vi "TA Main - PID - Copy.vi"() -> ()   [LabVIEW 2019]
doc: "This example demonstrates how to acquire a continuous amount of data (Waveform) using the DAQ device's internal clock. It also shows how to synchronize two devices for different device families (E Series, S Series, M Series, X Series, DSA, and SC Express), to simultaneously acquire the data.\n\nFor instructions on how to connect your signals to the DAQ device, refer to your device documentation."
uses:
  Program Files/National Instruments/LabVIEW 2019/examples/Instrument IO/Serial/support/Serial - Settings.ctl
  <vilib>/Utility/error.llb/DialogType.ctl
  <vilib>/DAQmx/read.llb/DAQmx Read (Analog 1D Wfm NChan NSamp).vi
  <vilib>/DAQmx/write.llb/DAQmx Write (Analog Wfm 1Chan NSamp).vi
  <vilib>/Instr/_visa.llb/VISA Configure Serial Port (Instr).vi
  <vilib>/DAQmx/configure/timing.llb/DAQmx Timing (Sample Clock).vi
  <vilib>/DAQmx/miscellaneous.llb/DAQmx Fill In Error Info.vi
panel:
  out "Heater Modulation":waveform(dbl)(graph)={"t0"=timestamp(28 s since 1904-01-01), "dt"=0.0001, "Y"=array[10000 elements]} caption="Waveform"
  out "Lockin chart 2":waveform(dbl)[](graph)=[{"t0"=timestamp(3657170606.5589848 s since 1904-01-01), "dt"=1.9999999999999998, "Y"=[-0.10259103252348788], "attributes"=variant("NI_ChannelName"=variant(string "Phase - Diode Voltage"), "NI_UnitDescription"=variant(string "Rad"))}, {"t0"=timestamp(3657170606.5589848 s since 1904-01-01), "dt"=1.9999999999999998, "Y"=[0.08995683165578135], "attributes"=variant("NI_ChannelName"=variant(string "Amplitude - Diode Voltage"), "NI_UnitDescription"=variant(string "Volts"))}]
  in  "Pass Logger":T1(tab)=enum."PID"
  out "CO2 chart":waveform(dbl)[](graph)=[{"t0"=timestamp(3657170606.3978887 s since 1904-01-01), "dt"=0.0, "Y"=[817.0], "attributes"=variant("NI_ChannelName"=variant(string "SCD30 CO2"), "NI_UnitDescription"=variant(string "ppm"))}, {"t0"=timestamp(3657170606.3978887 s since 1904-01-01), "dt"=0.0, "Y"=[23.97], "attributes"=variant("NI_ChannelName"=variant(string "SCD30 Temp"), "NI_UnitDescription"=variant(string "C"))}, {"t0"=timestamp(3657170606.3978887 s since 1904-01-01), "dt"=0.0, "Y"=[36.92], "attributes"=variant("NI_ChannelName"=variant(string "SCD30 Humidity"), "NI_UnitDescription"=variant(string "%"))}, {"t0"=timestamp(3657170606.3978887 s since 1904-01-01), "dt"=0.0, "Y"=[23.25], "attributes"=variant("NI_ChannelName"=variant(string "BME680 Temp"), "NI_UnitDescription"=variant(string "C"))}, {"t0"=timestamp(3657170606.3978887 s since 1904-01-01), "dt"=0.0, "Y"=[1004.82], "attributes"=variant("NI_ChannelName"=variant(string "hPa"), "NI_UnitDescription"=variant(string "BME680 Pressure"))}, {"t0"=timestamp(3657170606.3978887 s since 1904-01-01), "dt"=0.0, "Y"=[39.65], "attributes"=variant("NI_ChannelName"=variant(string "BME680 Humidity"), "NI_UnitDescription"=variant(string "%"))}, {"t0"=timestamp(3657170606.3978887 s since 1904-01-01), "dt"=0.0, "Y"=[747.02], "attributes"=variant("NI_ChannelName"=variant(string "BME680 Gas"), "NI_UnitDescription"=variant(string "KOhms"))}]
  in  "Stop":bool
  in  "Enable logging":bool caption="Enable"
  in  "File config":T2={"Filepath"=path "C:/Users/Administrator/Desktop/DAQ PAS/Test data", "Test ID"="test", "PC"="69DTQV2"}
  out "Lockin chart":waveform(dbl)[](graph)=[{"t0"=timestamp(3657170606.5589848 s since 1904-01-01), "dt"=1.9999999999999998, "Y"=[0.35840409569864184], "attributes"=variant("NI_ChannelName"=variant(string "Phase - Mic Diff"), "NI_UnitDescription"=variant(string "Rad"))}, {"t0"=timestamp(3657170606.5589848 s since 1904-01-01), "dt"=1.9999999999999998, "Y"=[0.04132909262078132], "attributes"=variant("NI_ChannelName"=variant(string "Amplitude - Mic Diff"), "NI_UnitDescription"=variant(string "Volts"))}]
  out "Lockin output 1":T3={"X"=0.01935147614577424, "Y"=0.007248713347471455, "R"=0.02066454631039066, "θ"=0.35840409569864184, "Amp"=0.04132909262078132, "dt"=1.9999999999999998, "Active channel"="Mic Diff", "Ref channel"="Heater Voltage"} {"X" format="%#_3g"; "Y" format="%#_3g"; "R" format="%#_3g"}
  out "Reference sesnsor readings":T4={"SCD30 CO2"=817.0, "SCD30 Temp (C)"=23.97, "SCD30 RH (%)"=36.92, "BME680 Temp (C) "=23.25, "BME680 Presssure (hPa)"=1004.82, "BME680 RH (%) "=39.65, "BME680 Gas (KOhms)"=747.02}
  in  "Sampling config":cluster{"Fs":dbl, "#s":dbl}={"Fs"=10000.0, "#s"=10000.0} {"Fs" format="%.2p"}
  in  "buffer size (in samples per channel)":u32
  in  "Config 1":cluster{"Ref Index":i32, "Active Index":i32}={"Ref Index"=2, "Active Index"=5}
  out "Lockin output 5":T3={"X"=-4.71813339906535, "Y"=-2.4285894180439636, "R"=5.306489360472804, "θ"=-2.66622648098918, "Amp"=10.612978720945607, "dt"=1.9999999999999998, "Active channel"="Heater Current", "Ref channel"="Heater Voltage"} {"X" format="%#_3g"; "Y" format="%#_3g"; "R" format="%#_3g"}
  out "Lockin output 6":T3={"X"=19.611612959634517, "Y"=6.527769643575472, "R"=20.66947361202239, "θ"=0.3213175235280957, "Amp"=41.33894722404478, "dt"=1.9999999999999998, "Active channel"="Heater Temperature", "Ref channel"="Heater Voltage"} {"X" format="%#_3g"; "Y" format="%#_3g"; "R" format="%#_3g"}
  out "Lockin output 4":T3={"X"=-0.22804529541896595, "Y"=-0.10244301108706262, "R"=0.24999845456183822, "θ"=-2.719385728324672, "Amp"=0.49999690912367645, "dt"=1.9999999999999998, "Active channel"="Heater Voltage", "Ref channel"="Heater Voltage"} {"X" format="%#_3g"; "Y" format="%#_3g"; "R" format="%#_3g"}
  out "Lockin output 3":T3={"X"=0.019485539557515245, "Y"=0.00689470931901729, "R"=0.02066937997234642, "θ"=0.34008918758761303, "Amp"=0.04133875994469284, "dt"=1.9999999999999998, "Active channel"="Mic Active", "Ref channel"="Heater Voltage"} {"X" format="%#_3g"; "Y" format="%#_3g"; "R" format="%#_3g"}
  out "Lockin output 2":T3={"X"=0.0003267413461158994, "Y"=-0.0008339623352990468, "R"=0.0008956858176610087, "θ"=-1.197384139538272, "Amp"=0.0017913716353220174, "dt"=1.9999999999999998, "Active channel"="Mic Ref", "Ref channel"="Heater Voltage"} {"X" format="%#_3g"; "Y" format="%#_3g"; "R" format="%#_3g"}
  in  "Config 5":cluster{"Ref Index":i32, "Active Index":i32}={"Ref Index"=2, "Active Index"=6}
  in  "Config 4":cluster{"Ref Index":i32, "Active Index":i32}={"Ref Index"=2, "Active Index"=2}
  in  "Config 3":cluster{"Ref Index":i32, "Active Index":i32}={"Ref Index"=2, "Active Index"=1}
  in  "Config 2":cluster{"Ref Index":i32, "Active Index":i32}={"Ref Index"=2, "Active Index"=0}
  in  "Config 6":cluster{"Ref Index":i32, "Active Index":i32}={"Ref Index"=2, "Active Index"=8}
  out "Lockin output 1":T3={"X"=0.01935147614577424, "Y"=0.007248713347471455, "R"=0.02066454631039066, "θ"=0.35840409569864184, "Amp"=0.04132909262078132, "dt"=1.9999999999999998, "Active channel"="Mic Diff", "Ref channel"="Heater Voltage"} {"X" format="%#_3g"; "Y" format="%#_3g"; "R" format="%#_3g"}
  in  "Config 7":cluster{"Ref Index":i32, "Active Index":i32}={"Ref Index"=2, "Active Index"=7}
  out "Lockin output 7":T3={"X"=-4.88093610591512, "Y"=-2.2652620290193846, "R"=5.3809803317000595, "θ"=-2.7070719289824767, "Amp"=10.761960663400119, "dt"=1.9999999999999998, "Active channel"="Heater Power", "Ref channel"="Heater Voltage"} {"X" format="%#_3g"; "Y" format="%#_3g"; "R" format="%#_3g"}
  in  "Config 8":cluster{"Ref Index":i32, "Active Index":i32}={"Ref Index"=2, "Active Index"=3}
  in  "Config 9":cluster{"Ref Index":i32, "Active Index":i32}={"Ref Index"=2, "Active Index"=4}
  out "Lockin output 9":T3={"X"=0.04474192624345704, "Y"=-0.004606292045853832, "R"=0.04497841582789067, "θ"=-0.10259103252348788, "Amp"=0.08995683165578135, "dt"=1.9999999999999998, "Active channel"="Diode Voltage", "Ref channel"="Heater Voltage"} {"X" format="%#_3g"; "Y" format="%#_3g"; "R" format="%#_3g"}
  out "Lockin output 8":T3={"X"=-0.04777429539770218, "Y"=-0.02309761120753558, "R"=0.0530648937080004, "θ"=-2.6912533488681167, "Amp"=0.1061297874160008, "dt"=1.9999999999999998, "Active channel"="Heater Shunt", "Ref channel"="Heater Voltage"} {"X" format="%#_3g"; "Y" format="%#_3g"; "R" format="%#_3g"}
  in  "VISA resource name 2":refnum<visa-resource-name>="COM6"
  in  "Serial Settings":T5={"baud rate"=9600, "data bits"=8, "parity"=enum."None", "stop bits"=10, "flow control"=0} {"flow control" items=["None"=0, "XON/XOFF"=1, "RTS/CTS"=2, "DTR/DSR"=4]; "stop bits" items=["1.0"=10, "1.5"=15, "2.0"=20]; "data bits" min=5 max=8 step=1; "baud rate" items=["75"=75, "110"=110, "134"=134, "150"=150, "300"=300, "600"=600, "1200"=1200, "1800"=1800, "2400"=2400, "4800"=4800, "7200"=7200, "9600"=9600, "14400"=14400, "19200"=19200, "28800"=28800, "38400"=38400, "56000"=56000, "57600"=57600, "115200"=115200, "128000"=128000, "230400"=230400]}
  out "Waveform":waveform(dbl)(graph)={"t0"=timestamp(3657170606.558974 s since 1904-01-01), "dt"=9.999999999999999e-05, "Y"=array[20001 elements], "attributes"=variant("NI_ChannelName"=variant(string "Mic Diff"), "NI_UnitDescription"=variant(string "Volts"))}
  in  "Config":T6={"Active Index"=1, "Ref Index"=0, "Gain"=1.0, "Channel name"="Mic Diff", "Enable"=TRUE, "Offset"=0.0}
  out "Channel names":T7={"Active channel"="Mic Active", "Ref channel"="Mic Ref"}
  in  "Waveform Config":T8={"Frequency"=10.0, "Voltage (V)"=1.0, "Signal type"=enum."Sine Wave", "Square wave duty cycle (%)"=50.0, "Offset (V)"=0.0, "DC shift"=TRUE} {"Square wave duty cycle (%)" format="%0.2f"}
  in  "Output range":cluster{"output high":dbl, "output low":dbl}={"output high"=1.6, "output low"=0.0}
  in  "Channel config":T9={"physical channels"="Dev1/ao0", "name to assign"="Heater Voltage"}
  in  "Config":T10={"Voltage channel index"=2, "Shunt channel index"=3, "Shunt resistance"=10}
  out "Channel names":T11={"Voltage channel name"="Heater Voltage", "Shunt channel name"="Heater Shunt"}
  out "Microphone Waveform":waveform(dbl)[](graph)=[{"t0"=timestamp(3657170606.558963 s since 1904-01-01), "dt"=9.999999999999999e-05, "Y"=array[20001 elements], "attributes"=variant("NI_ChannelName"=variant(string "Mic Ref"), "NI_UnitDescription"=variant(string "Volts"))}, {"t0"=timestamp(3657170606.558974 s since 1904-01-01), "dt"=9.999999999999999e-05, "Y"=array[20001 elements], "attributes"=variant("NI_ChannelName"=variant(string "Mic Active"), "NI_UnitDescription"=variant(string "Volts"))}, {"t0"=timestamp(3657170606.5589848 s since 1904-01-01), "dt"=9.999999999999999e-05, "Y"=array[20001 elements], "attributes"=variant("NI_ChannelName"=variant(string "Heater Voltage"), "NI_UnitDescription"=variant(string "Volts"))}, {"t0"=timestamp(3657170606.5589957 s since 1904-01-01), "dt"=9.999999999999999e-05, "Y"=array[20001 elements], "attributes"=variant("NI_ChannelName"=variant(string "Heater Shunt"), "NI_UnitDescription"=variant(string "Volts"))}, {"t0"=timestamp(3657170606.5590067 s since 1904-01-01), "dt"=9.999999999999999e-05, "Y"=array[20001 elements], "attributes"=variant("NI_ChannelName"=variant(string "Diode Voltage"), "NI_UnitDescription"=variant(string "Volts"))}, {"t0"=timestamp(3657170606.558974 s since 1904-01-01), "dt"=9.999999999999999e-05, "Y"=array[20001 elements], "attributes"=variant("NI_ChannelName"=variant(string "Mic Diff"), "NI_UnitDescription"=variant(string "Volts"))}, {"t0"=timestamp(3657170606.5589957 s since 1904-01-01), "dt"=9.999999999999999e-05, "Y"=array[20001 elements], "attributes"=variant("NI_ChannelName"=variant(string "Heater Current"), "NI_UnitDescription"=variant(string "mA"))}, {"t0"=timestamp(3657170606.5589848 s since 1904-01-01), "dt"=9.999999999999999e-05, "Y"=array[20001 elements], "attributes"=variant("NI_ChannelName"=variant(string "Heater Power"), "NI_UnitDescription"=variant(string "mW"))}, {"t0"=timestamp(3657170606.558974 s since 1904-01-01), "dt"=9.999999999999999e-05, "Y"=array[20001 elements], "attributes"=variant("NI_ChannelName"=variant(string "Heater Temperature"), "NI_UnitDescription"=variant(string "degC"))}]
  out "Heater Waveform":waveform(dbl)[](graph)=[{"t0"=timestamp(3657170606.558963 s since 1904-01-01), "dt"=9.999999999999999e-05, "Y"=array[20001 elements], "attributes"=variant("NI_ChannelName"=variant(string "Mic Ref"), "NI_UnitDescription"=variant(string "Volts"))}, {"t0"=timestamp(3657170606.558974 s since 1904-01-01), "dt"=9.999999999999999e-05, "Y"=array[20001 elements], "attributes"=variant("NI_ChannelName"=variant(string "Mic Active"), "NI_UnitDescription"=variant(string "Volts"))}, {"t0"=timestamp(3657170606.5589848 s since 1904-01-01), "dt"=9.999999999999999e-05, "Y"=array[20001 elements], "attributes"=variant("NI_ChannelName"=variant(string "Heater Voltage"), "NI_UnitDescription"=variant(string "Volts"))}, {"t0"=timestamp(3657170606.5589957 s since 1904-01-01), "dt"=9.999999999999999e-05, "Y"=array[20001 elements], "attributes"=variant("NI_ChannelName"=variant(string "Heater Shunt"), "NI_UnitDescription"=variant(string "Volts"))}, {"t0"=timestamp(3657170606.5590067 s since 1904-01-01), "dt"=9.999999999999999e-05, "Y"=array[20001 elements], "attributes"=variant("NI_ChannelName"=variant(string "Diode Voltage"), "NI_UnitDescription"=variant(string "Volts"))}, {"t0"=timestamp(3657170606.558974 s since 1904-01-01), "dt"=9.999999999999999e-05, "Y"=array[20001 elements], "attributes"=variant("NI_ChannelName"=variant(string "Mic Diff"), "NI_UnitDescription"=variant(string "Volts"))}, {"t0"=timestamp(3657170606.5589957 s since 1904-01-01), "dt"=9.999999999999999e-05, "Y"=array[20001 elements], "attributes"=variant("NI_ChannelName"=variant(string "Heater Current"), "NI_UnitDescription"=variant(string "mA"))}, {"t0"=timestamp(3657170606.5589848 s since 1904-01-01), "dt"=9.999999999999999e-05, "Y"=array[20001 elements], "attributes"=variant("NI_ChannelName"=variant(string "Heater Power"), "NI_UnitDescription"=variant(string "mW"))}, {"t0"=timestamp(3657170606.558974 s since 1904-01-01), "dt"=9.999999999999999e-05, "Y"=array[20001 elements], "attributes"=variant("NI_ChannelName"=variant(string "Heater Temperature"), "NI_UnitDescription"=variant(string "degC"))}]
  out "Diode Waveform":waveform(dbl)[](graph)=[{"t0"=timestamp(3657170606.558963 s since 1904-01-01), "dt"=9.999999999999999e-05, "Y"=array[20001 elements], "attributes"=variant("NI_ChannelName"=variant(string "Mic Ref"), "NI_UnitDescription"=variant(string "Volts"))}, {"t0"=timestamp(3657170606.558974 s since 1904-01-01), "dt"=9.999999999999999e-05, "Y"=array[20001 elements], "attributes"=variant("NI_ChannelName"=variant(string "Mic Active"), "NI_UnitDescription"=variant(string "Volts"))}, {"t0"=timestamp(3657170606.5589848 s since 1904-01-01), "dt"=9.999999999999999e-05, "Y"=array[20001 elements], "attributes"=variant("NI_ChannelName"=variant(string "Heater Voltage"), "NI_UnitDescription"=variant(string "Volts"))}, {"t0"=timestamp(3657170606.5589957 s since 1904-01-01), "dt"=9.999999999999999e-05, "Y"=array[20001 elements], "attributes"=variant("NI_ChannelName"=variant(string "Heater Shunt"), "NI_UnitDescription"=variant(string "Volts"))}, {"t0"=timestamp(3657170606.5590067 s since 1904-01-01), "dt"=9.999999999999999e-05, "Y"=array[20001 elements], "attributes"=variant("NI_ChannelName"=variant(string "Diode Voltage"), "NI_UnitDescription"=variant(string "Volts"))}, {"t0"=timestamp(3657170606.558974 s since 1904-01-01), "dt"=9.999999999999999e-05, "Y"=array[20001 elements], "attributes"=variant("NI_ChannelName"=variant(string "Mic Diff"), "NI_UnitDescription"=variant(string "Volts"))}, {"t0"=timestamp(3657170606.5589957 s since 1904-01-01), "dt"=9.999999999999999e-05, "Y"=array[20001 elements], "attributes"=variant("NI_ChannelName"=variant(string "Heater Current"), "NI_UnitDescription"=variant(string "mA"))}, {"t0"=timestamp(3657170606.5589848 s since 1904-01-01), "dt"=9.999999999999999e-05, "Y"=array[20001 elements], "attributes"=variant("NI_ChannelName"=variant(string "Heater Power"), "NI_UnitDescription"=variant(string "mW"))}, {"t0"=timestamp(3657170606.558974 s since 1904-01-01), "dt"=9.999999999999999e-05, "Y"=array[20001 elements], "attributes"=variant("NI_ChannelName"=variant(string "Heater Temperature"), "NI_UnitDescription"=variant(string "degC"))}]
  in  "Channel 4 config":T12={"Channel"="Dev1/ai3", "Vmax"=0.5, "Vmin"=0.0, "name to assign"="Heater Shunt", "input terminal configuration"=10106} {"input terminal configuration" items=["Default"=-1, "RSE"=10083, "NRSE"=10078, "Differential"=10106, "Pseudodifferential"=12529]; "Vmin" format="%0.2f"; "Vmax" format="%0.2f"}
  in  "Channel 3 config":T12={"Channel"="Dev1/ai2", "Vmax"=3.0, "Vmin"=0.0, "name to assign"="Heater Voltage", "input terminal configuration"=10083} {"input terminal configuration" items=["Default"=-1, "RSE"=10083, "NRSE"=10078, "Differential"=10106, "Pseudodifferential"=12529]; "Vmin" format="%0.2f"; "Vmax" format="%0.2f"}
  in  "Channel 2 config":T12={"Channel"="Dev1/ai1", "Vmax"=3.0, "Vmin"=-3.0, "name to assign"="Mic Active", "input terminal configuration"=10083} {"input terminal configuration" items=["Default"=-1, "RSE"=10083, "NRSE"=10078, "Differential"=10106, "Pseudodifferential"=12529]; "Vmin" format="%0.2f"; "Vmax" format="%0.2f"}
  in  "Channel 1 config":T12={"Channel"="Dev1/ai0", "Vmax"=3.0, "Vmin"=-3.0, "name to assign"="Mic Ref", "input terminal configuration"=10083} {"input terminal configuration" items=["Default"=-1, "RSE"=10083, "NRSE"=10078, "Differential"=10106, "Pseudodifferential"=12529]; "Vmin" format="%0.2f"; "Vmax" format="%0.2f"}
  in  "Channel 5 config":T12={"Channel"="Dev1/ai4", "Vmax"=1.0, "Vmin"=0.0, "name to assign"="Diode Voltage", "input terminal configuration"=10083} {"input terminal configuration" items=["Default"=-1, "RSE"=10083, "NRSE"=10078, "Differential"=10106, "Pseudodifferential"=12529]; "Vmin" format="%0.2f"; "Vmax" format="%0.2f"}
  out "Boolean":bool
  out "PID output":dbl format="%.2f"
  in  "reinitialize? (F)":bool
  in  "auto? (F)":bool
  in  "PID gains":T13={"proportional gain (Kc)"=0.0125026, "integral time (Ti, min)"=2.0, "derivative time (Td, min)"=0.0} {"derivative time (Td, min)" format="%.6f"; "integral time (Ti, min)" format="%.6f"; "proportional gain (Kc)" format="%.6f"}
  in  "Temp config":T14={"Channel Index"=4, "TC"=0.001, "Channel name"="Heater Temperature", "25C Voltage"=0.80857} {"25C Voltage" format="%.5f"; "TC" format="%#_6f"}
  out "Sensor channel":string="Mic Active"
  in  "Store":bool
  in  "setpoint":dbl
  # "PAS Logger"
  # "(ppm)"
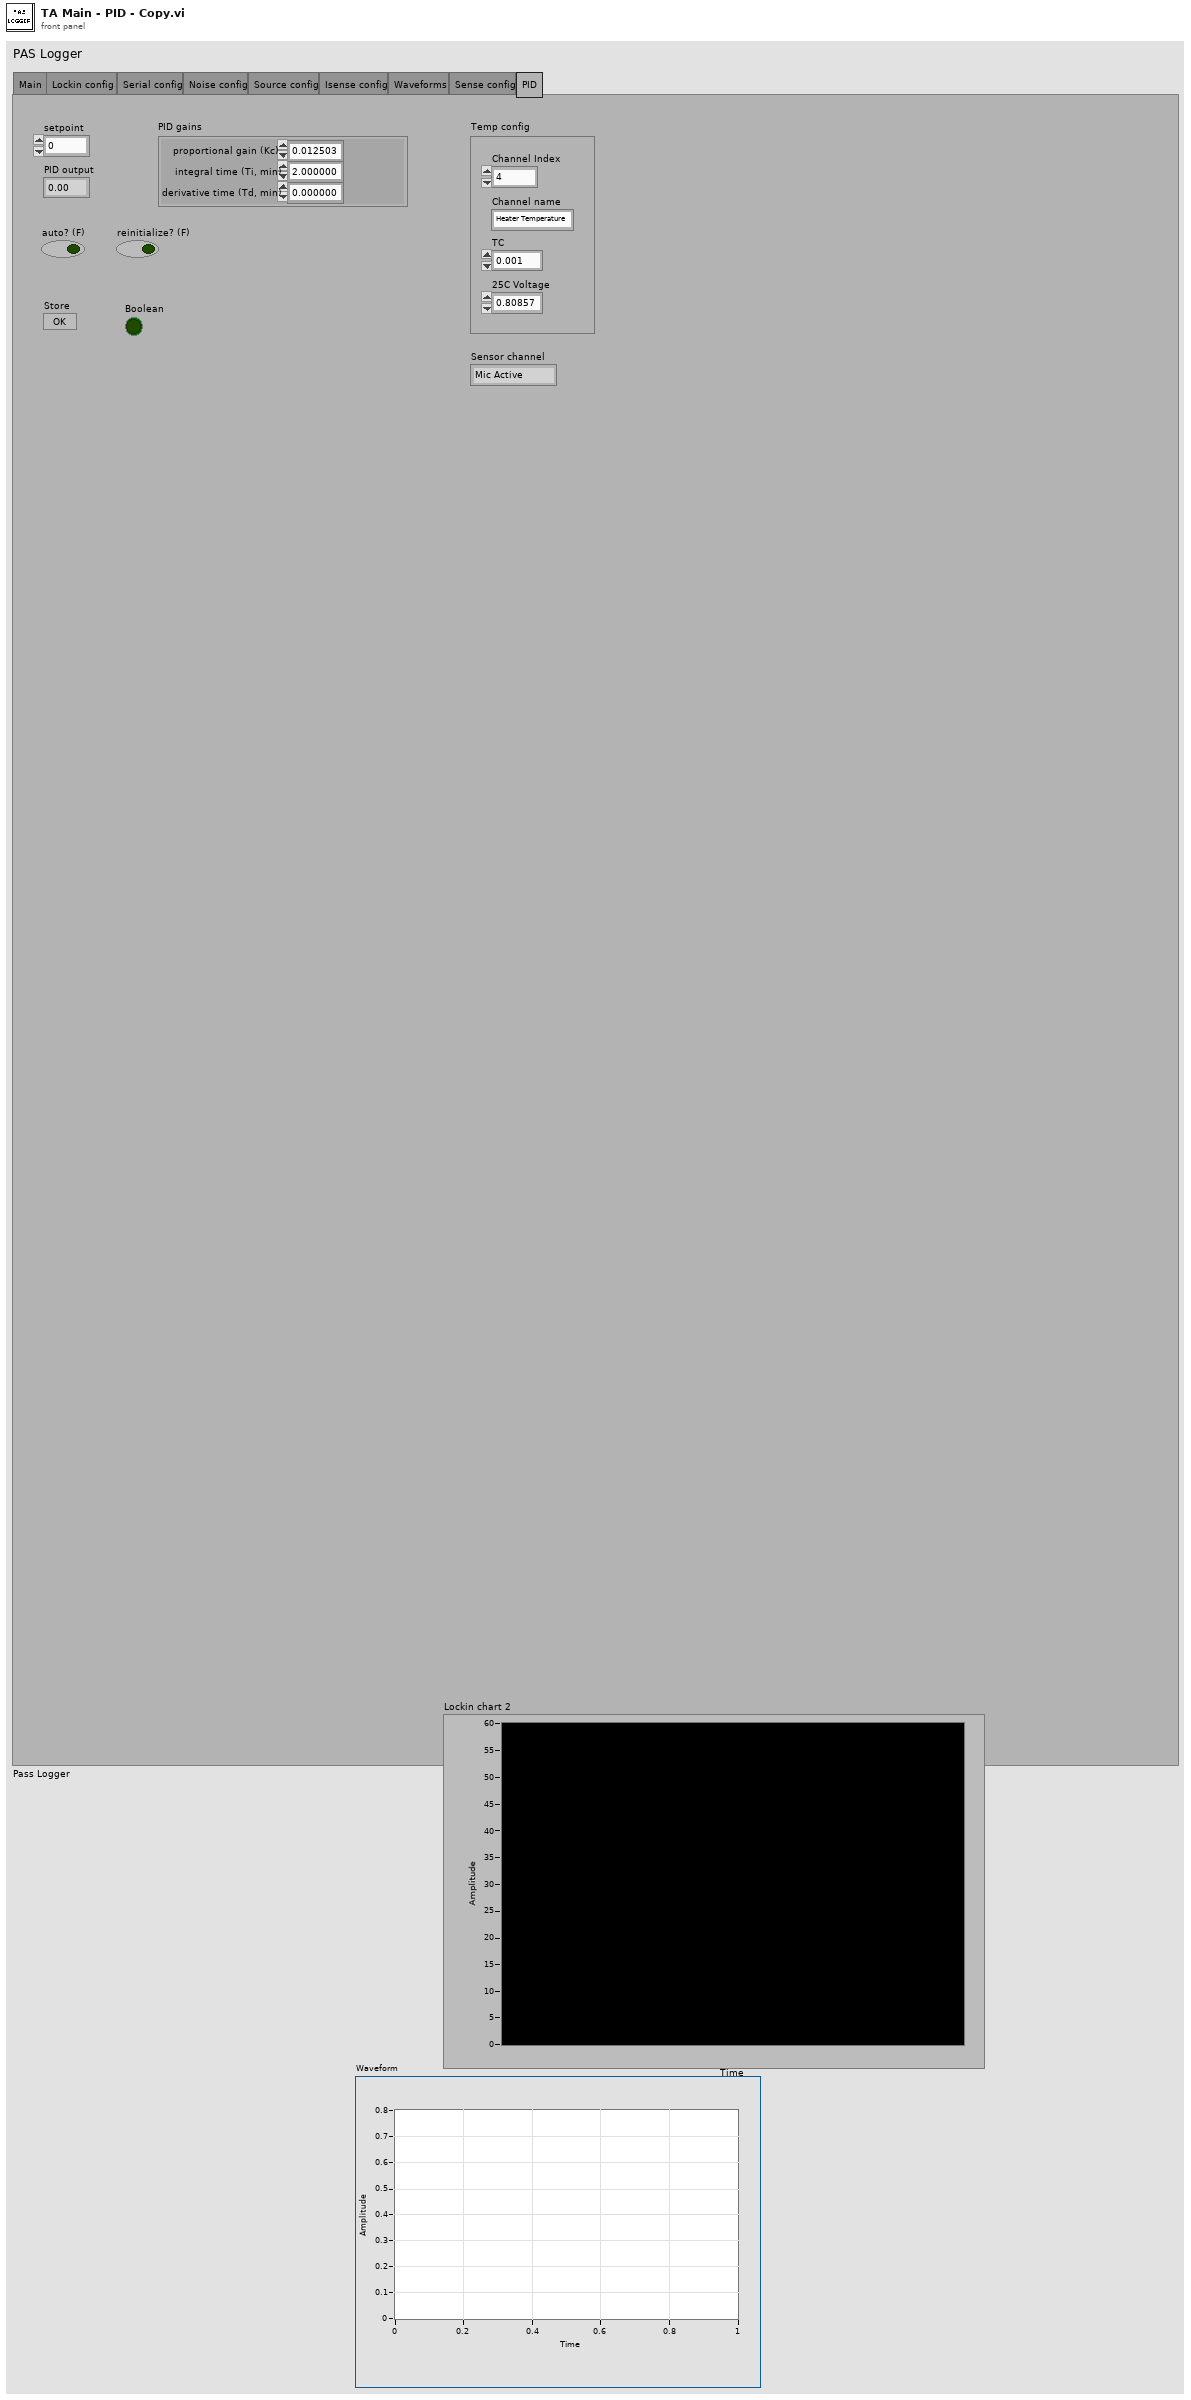
[diagram p1: front panel]
types:
  T1 = enum32{"Main", "Lockin config", "Serial config", "Noise config", "Source config", "Isense config", "Waveforms", "Sense config", "PID"}
  T2 = cluster{"Filepath":path, "Test ID":string, "PC":string}
  T3 = cluster{"X":dbl, "Y":dbl, "R":dbl, "θ":dbl, "Amp":dbl, "dt":dbl, "Active channel":string, "Ref channel":string}
  T4 = cluster{"SCD30 CO2":dbl, "SCD30 Temp (C)":dbl, "SCD30 RH (%)":dbl, "BME680 Temp (C) ":dbl, "BME680 Presssure (hPa)":dbl, "BME680 RH (%) ":dbl, "BME680 Gas (KOhms)":dbl}
  T5 = typedef "Serial - Settings.ctl" = cluster{"baud rate":u32, "data bits":u16, "parity":enum16{"None", "Odd", "Even", "Mark", "Space"}, "stop bits":u16, "flow control":u16}
  T6 = cluster{"Active Index":i32, "Ref Index":i32, "Gain":dbl, "Channel name":string, "Enable":bool, "Offset":dbl}
  T7 = cluster{"Active channel":string, "Ref channel":string}
  T8 = cluster{"Frequency":dbl, "Voltage (V)":dbl, "Signal type":enum16{"Sine Wave", "Triangle Wave", "Square Wave", "Sawtooth Wave"}, "Square wave duty cycle (%)":dbl, "Offset (V)":dbl, "DC shift":bool}
  T9 = cluster{"physical channels":tag, "name to assign":string}
  T10 = cluster{"Voltage channel index":i32, "Shunt channel index":i32, "Shunt resistance":i32}
  T11 = cluster{"Voltage channel name":string, "Shunt channel name":string}
  T12 = cluster{"Channel":tag, "Vmax":dbl, "Vmin":dbl, "name to assign":string, "input terminal configuration":i32}
  T13 = cluster{"proportional gain (Kc)":dbl, "integral time (Ti, min)":dbl, "derivative time (Td, min)":dbl}
  T14 = cluster{"Channel Index":i32, "TC":dbl, "Channel name":string, "25C Voltage":dbl}
  T15 = typedef "DialogType.ctl" = u16
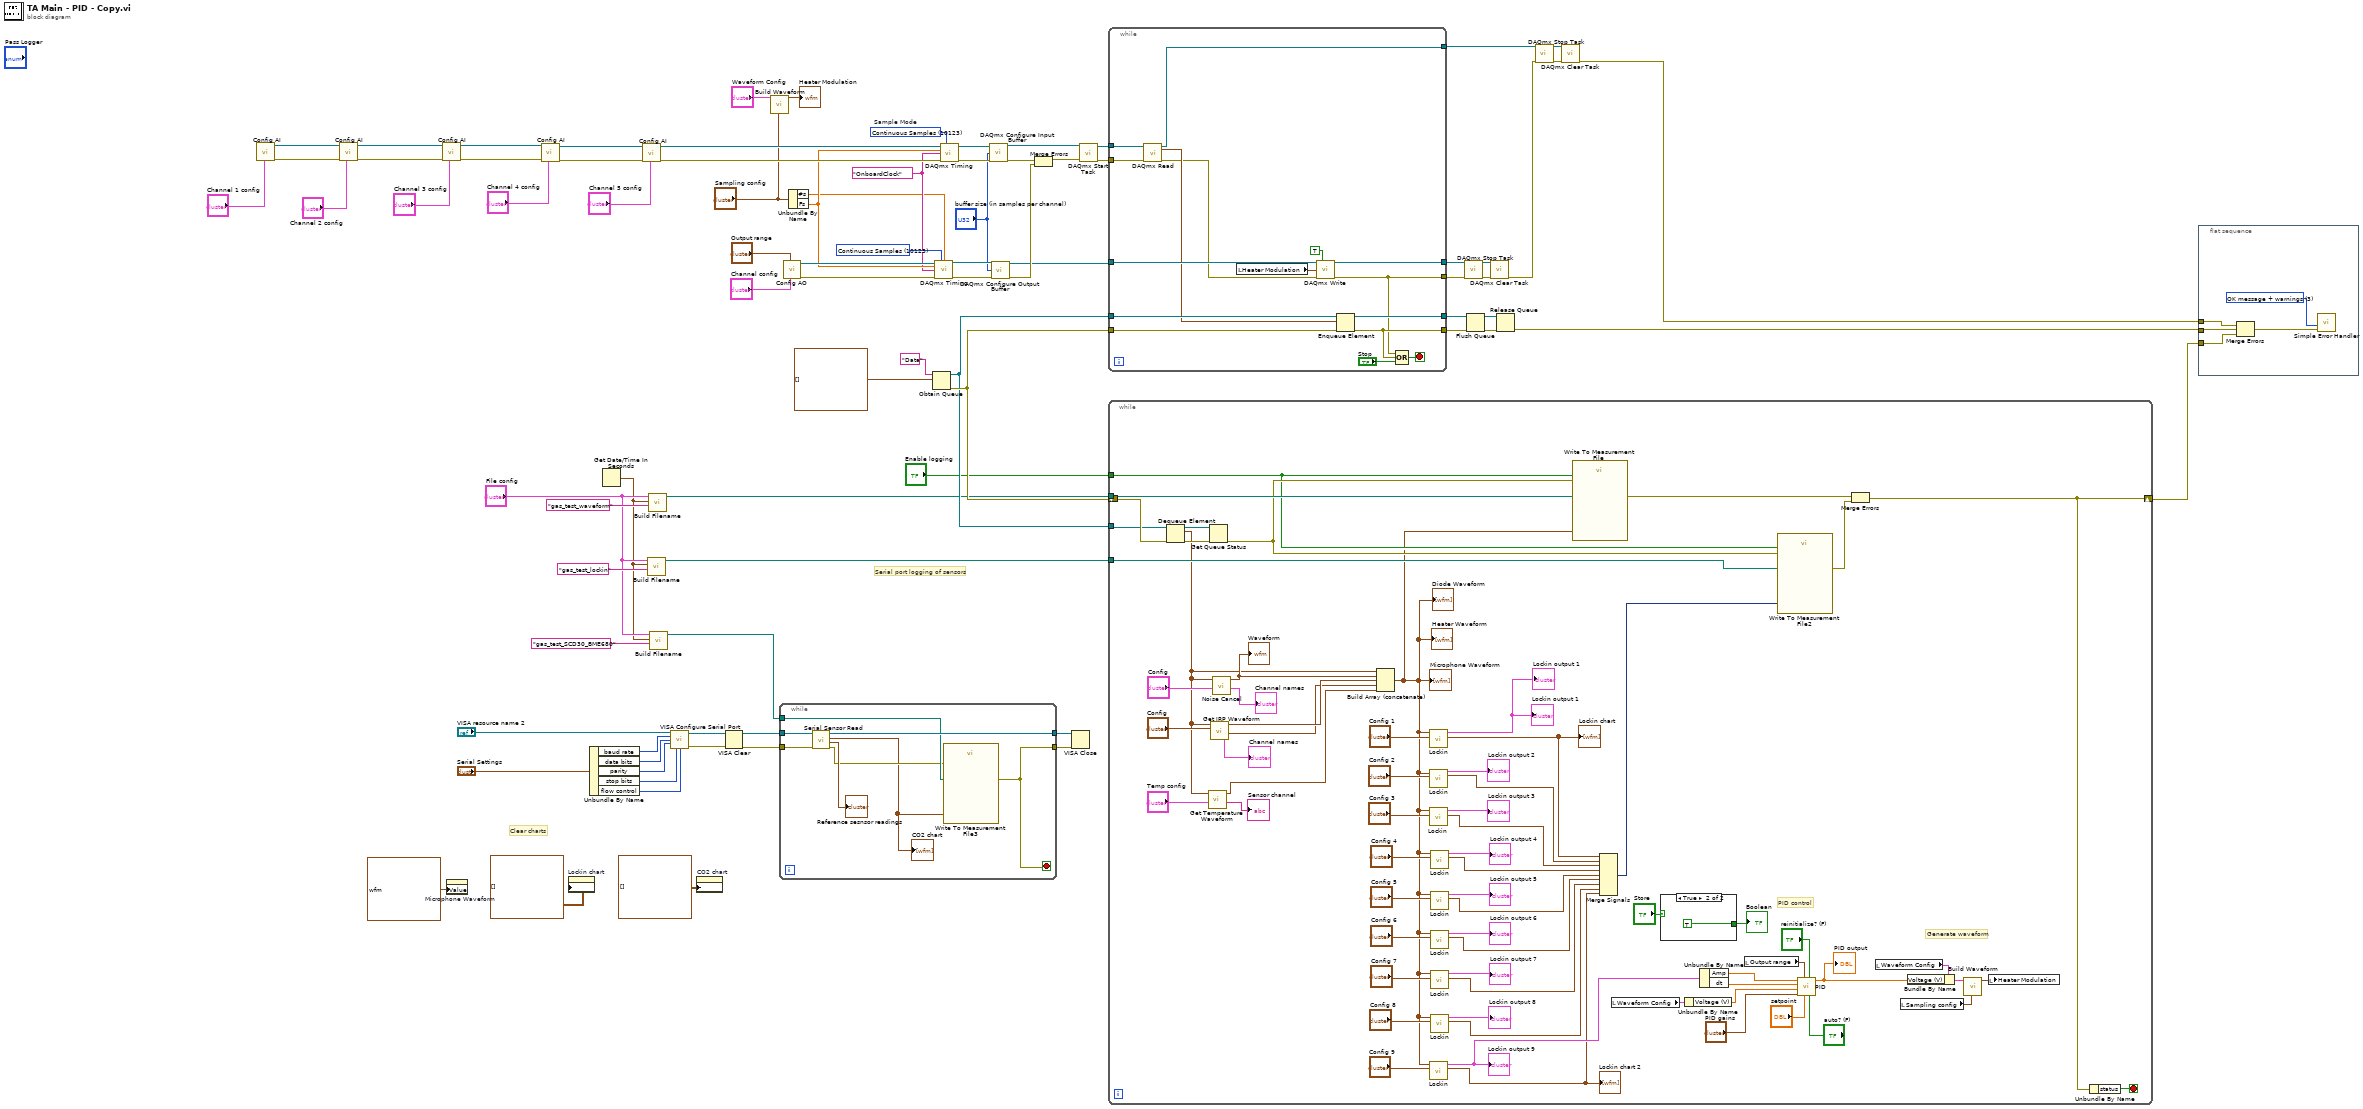
[diagram p0: block diagram]
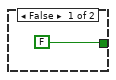
[diagram p2: hidden frame]
diagram:
  w32 = 10123 items=["Finite Samples"=10178, "Continuous Samples"=10123, "Hardware Timed Single Point"=12522] ("sample mode")
  w26 = tag "OnboardClock" ("source")
  w81 = 10123 items=["Finite Samples"=10178, "Continuous Samples"=10123, "Hardware Timed Single Point"=12522]  # Sample Mode
  # "Clear charts"
  # "Serial port logging of sensors"
  n1 = call "Config AI.vi"("Channel config"="Channel 1 config") -> ("error out"=w80:errorcluster, "task out"=w79:refnum<k21>)  [unwired: 9 in]
  n2 = call "Config AI.vi"("Channel config"="Channel 2 config", "error in"=w80, "task in"=w79) -> ("error out"=w37:errorcluster, "task out"=w36:refnum<k21>)  [unwired: 7 in]
  n3 = call "Config AI.vi"("Channel config"="Channel 3 config", "error in"=w37, "task in"=w36) -> ("error out"=w68:errorcluster, "task out"=w67:refnum<k21>)  [unwired: 7 in]
  n4 = property on="Microphone Waveform" class="WFGraph (strict)"("Value"=waveform(dbl)[] [{"t0"=timestamp(3651561790.263236 s since 1904-01-01), "dt"=0.001, "Y"=array[2000 elements], "attributes"=variant("NI_ChannelName"=variant(string "Mic Active"), "NI_UnitDescription"=variant(string "Volts"))}, {"t0"=timestamp(3651561790.263247 s since 1904-01-01), "dt"=0.001, "Y"=array[2000 elements], "attributes"=variant("NI_ChannelName"=variant(string "Mic Ref"), "NI_UnitDescription"=variant(string "Volts"))}, {"t0"=timestamp(3651561790.263258 s since 1904-01-01), "dt"=0.001, "Y"=array[2000 elements], "attributes"=variant("NI_ChannelName"=variant(string "Diode Heater"), "NI_UnitDescription"=variant(string "Volts"))}, {"t0"=timestamp(3651561790.263269 s since 1904-01-01), "dt"=0.001, "Y"=array[2000 elements], "attributes"=variant("NI_ChannelName"=variant(string "Diode Amb"), "NI_UnitDescription"=variant(string "Volts"))}, {"t0"=timestamp(3651561790.26328 s since 1904-01-01), "dt"=0.001, "Y"=array[2000 elements], "attributes"=variant("NI_ChannelName"=variant(string "Heater Shunt"), "NI_UnitDescription"=variant(string "Volts"))}, {"t0"=timestamp(3651561790.2632914 s since 1904-01-01), "dt"=0.001, "Y"=array[2000 elements], "attributes"=variant("NI_ChannelName"=variant(string "Heater V"), "NI_UnitDescription"=variant(string "Volts"))}, {"t0"=timestamp(3651561790.263247 s since 1904-01-01), "dt"=0.001, "Y"=array[2000 elements], "attributes"=variant("NI_ChannelName"=variant(string "Mic Diff"), "NI_UnitDescription"=variant(string "Volts"))}, {"t0"=timestamp(3651561790.26328 s since 1904-01-01), "dt"=0.001, "Y"=array[2000 elements], "attributes"=variant("NI_ChannelName"=variant(string "Heater Current"), "NI_UnitDescription"=variant(string "Amps"))}] ("Waveform")) -> ()  [unwired: 2 in, 2 out]
  n5 = call "Config AI.vi"("Channel config"="Channel 4 config", "error in"=w68, "task in"=w67) -> ("error out"=w34:errorcluster, "task out"=w33:refnum<k21>)  [unwired: 7 in]
  n6 = property on="Lockin chart" class="WFChart (strict)"("History Data"=waveform(dbl)[][] []) -> ()  [unwired: 2 in, 2 out]
  n7 = Unbundle By Name("Serial Settings") -> ("baud rate"=w52:u32, "data bits"=w51:u16, "parity"=w50:enum16{"None", "Odd", "Even", "Mark", "Space"}, "stop bits"=w49:u16, "flow control"=w48:u16)
  n8 = Get Date/Time In Seconds() -> (seconds since 1Jan1904=w55:timestamp)
  n9 = call "Config AI.vi"("Channel config"="Channel 5 config", "error in"=w34, "task in"=w33) -> ("error out"=w29:errorcluster, "task out"=w28:refnum<k21>)  [unwired: 7 in]
  n10 = call "Build Filename.vi"("Test type"="gas_test_lockin" ("File Descriptor"), "time stamp"=w55, "File config"="File config") -> ("appended path"=w58:path)  [unwired: 8 in]
  n11 = call "Build Filename.vi"("Test type"="gas_test_waveform" ("File type"), "time stamp"=w55, "File config"="File config") -> ("appended path"=w60:path)  [unwired: 8 in]
  n12 = call "Build Filename.vi"("Test type"="gas_test_SCD30_BME680" ("File Descriptor"), "time stamp"=w55, "File config"="File config") -> ("appended path"=w41:path)  [unwired: 8 in]
  n13 = call-poly "VISA Configure Serial Port"("VISA resource name"="VISA resource name 2", "baud rate (9600)"=w52, "data bits (8)"=w51, "parity (0:none)"=w50, "stop bits (10: 1 bit)"=w49, "flow control (0:none)"=w48) -> ("VISA resource name out"=w46:refnum<visa-resource-name>, "error out"=w47:errorcluster)  [unwired: 3 in, 5 out]
  n14 = property on="CO2 chart" class="WFChart (strict)"("History Data"=waveform(dbl)[][] []) -> ()  [unwired: 2 in, 2 out]
  n15 = VISA Clear(VISA resource name=w46, error in (no error)=w47) -> (VISA resource name out=w45:refnum<visa-resource-name>, error out=w44:errorcluster)
  n16 = call "Build Waveform.vi"("sampling config"="Sampling config", "Config"="Waveform Config") -> ("Waveform"=→"Heater Modulation":waveform(dbl))  [unwired: 8 in, 1 out]
  n17 = while {
    tunnel: w45 -> [w91]
    tunnel: w44 -> [w90]
    tunnel: [w85] -> w43
    tunnel: [w89] -> w42
    tunnel: w41 -> [w87]
    stop <- w85 stop-if-true
    n18 = call "Serial Sensor Read.vi"("error in (no error)"=w90, "VISA resource name"=w91) -> ("error out"=w86:errorcluster, "Readings"=→"Reference sesnsor readings":T4, "appended array"=w84:waveform(dbl)[], "VISA resource name out"=w89:refnum<visa-resource-name>)  [unwired: 6 in]
    "CO2 chart" <- w84
    n19 = call "Write To Measurement File3"("Signals"=w84, "error in (no error)"=w86, "Filename"=w87) -> ("error out"=w85:errorcluster)  [unwired: 14 in, 2 out]
  }
  n20 = call "Config AO.vi"("Channel config"="Channel config", "Output range"="Output range") -> ("error out"=w31:errorcluster, "task out"=w30:refnum<k21>)  [unwired: 8 in]
  n21 = Unbundle By Name("Sampling config") -> ("#s"=w15:dbl, "Fs"=w27:dbl)
  n22 = Obtain Queue(name (unnamed)="Data" ("名前（名前なし）"), element data type=waveform(dbl)[] [] ("data")) -> (queue out=w71:refnum<queue>, error out=w72:errorcluster)  [unwired: 3 in, 1 out]
  n23 = call-poly <vilib>:"DAQmx Timing.vi"("task/channels in"=w30, "sample mode"=w32, "samples per channel"=w15, "rate"=w27, "source"=w26, "error in"=w31) -> ("task out"=w5:refnum<k21>, "error out"=w4:errorcluster)  [unwired: 8 in]
  n24 = call-poly <vilib>:"DAQmx Timing.vi"("task/channels in"=w28, "sample mode"=w81, "rate"=w27, "source"=w26, "error in"=w29) -> ("task out"=w7:refnum<k21>, "error out"=w9:errorcluster)  [unwired: 9 in]
  n25 = call <vilib>:"DAQmx Configure Input Buffer.vi"("task/channels in"=w7, "buffer size (in samples per channel)"="buffer size (in samples per channel)", "error in"=w9) -> ("task out"=w6:refnum<k21>, "error out"=w8:errorcluster)  [unwired: 11 in]
  n26 = call <vilib>:"DAQmx Configure Output Buffer.vi"("task/channels in"=w5, "buffer size (in samples per channel)"="buffer size (in samples per channel)", "error in"=w4) -> ("task out"=w2:refnum<k21>, "error out"=w3:errorcluster)  [unwired: 11 in]
  n27 = Merge Errors(w8, w3) -> (w11:errorcluster)
  n28 = VISA Close(VISA resource name=w42, error in (no error)=w43) -> ()  [unwired: 1 out]
  n29 = call <vilib>:"DAQmx Start Task.vi"("task/channels in"=w6, "error in"=w11) -> ("task out"=w25:refnum<k21>, "error out"=w24:errorcluster)  [unwired: 12 in]
  n30 = while {
    tunnel: w71 -> [w158]
    shift-right: [w149] -> w70
    shift-left: w72 -> [w159]
    tunnel: w60 -> [w157]
    tunnel: "Enable logging" -> [w153]
    tunnel: w58 -> [w152]
    stop <- w145 stop-if-true
    # "Generate waveform"
    # "PID control"
    n31 = Dequeue Element(queue=w158, error in (no error)=w159) -> (queue out=w155:refnum<queue>, element=w114:waveform(dbl)[], error out=w156:errorcluster)  [unwired: 1 in, 1 out]
    n32 = call "Get Temperature Waveform.vi"("Config"="Temp config", "array"=w114) -> ("Channel name"=→"Sensor channel":string, "waveform out"=w111:waveform(dbl))  [unwired: 8 in]
    n33 = Get Queue Status(queue=w155, error in (no error)=w156) -> (error out=w154:errorcluster)  [unwired: 1 in, 7 out]
    n34 = call "Get IRP Waveform.vi"("Channel config"="Config", "array"=w114) -> ("Power waveform out"=w112:waveform(dbl), "Current waveform out"=w125:waveform(dbl), "Channel names"=→"Channel names":T11)  [unwired: 6 in, 1 out]
    n35 = call "Noise Cancel.vi"("Config"="Config", "array"=w114) -> ("Channel names"=→"Channel names":T7, "waveform out"=w147:waveform(dbl))  [unwired: 8 in]
    "Waveform" <- w147
    n36 = Build Array (concatenate)(w114, w147, w125, w112, w111) -> (w116:waveform(dbl)[])
    "Microphone Waveform" <- w116
    "Heater Waveform" <- w116
    "Diode Waveform" <- w116
    n37 = call "Lockin.vi"("Config"="Config 3", "array"=w116) -> ("Output waveform"=w142:waveform(dbl)[], "Lockin output"=→"Lockin output 3":T3)  [unwired: 8 in]
    n38 = call "Lockin.vi"("Config"="Config 1", "array"=w116) -> ("Output waveform"=w127:waveform(dbl)[], "Lockin output"=→"Lockin output 1" →"Lockin output 1":T3)  [unwired: 8 in]
    "Lockin chart" <- w127
    n39 = call "Lockin.vi"("Config"="Config 2", "array"=w116) -> ("Output waveform"=w143:waveform(dbl)[], "Lockin output"=→"Lockin output 2":T3)  [unwired: 8 in]
    n40 = call "Lockin.vi"("Config"="Config 9", "array"=w116) -> ("Output waveform"=w102:waveform(dbl)[], "Lockin output"=w104:T3)  [unwired: 8 in]
    "Lockin output 9" <- w104
    "Lockin chart 2" <- w102
    n41 = call "Lockin.vi"("Config"="Config 4", "array"=w116) -> ("Output waveform"=w141:waveform(dbl)[], "Lockin output"=→"Lockin output 4":T3)  [unwired: 8 in]
    n42 = call "Lockin.vi"("Config"="Config 8", "array"=w116) -> ("Output waveform"=w118:waveform(dbl)[], "Lockin output"=→"Lockin output 8":T3)  [unwired: 8 in]
    n43 = call "Lockin.vi"("Config"="Config 5", "array"=w116) -> ("Output waveform"=w140:waveform(dbl)[], "Lockin output"=→"Lockin output 5":T3)  [unwired: 8 in]
    n44 = call "Lockin.vi"("Config"="Config 6", "array"=w116) -> ("Output waveform"=w139:waveform(dbl)[], "Lockin output"=→"Lockin output 6":T3)  [unwired: 8 in]
    n45 = call "Lockin.vi"("Config"="Config 7", "array"=w116) -> ("Output waveform"=w121:waveform(dbl)[], "Lockin output"=→"Lockin output 7":T3)  [unwired: 8 in]
    n46 = call "Write To Measurement File"("Signals"=w116, "Enable"=w153, "error in (no error)"=w154, "Filename"=w157) -> ("error out"=w150:errorcluster)  [unwired: 13 in, 2 out]
    n47 = Merge Signals(w127, w143, w142, w141, w140, w139, w121, w118, w102) -> (w138:dynamicdata)
    n48 = local read "Waveform Config"() -> (w101:T8)
    n49 = case shown="True" "Store" {
      tunnel: [FALSE TRUE ("Boolean")] -> w92
      frame False {
      }
      frame True {
      }
    }
    "Boolean" <- w92
    n50 = Unbundle By Name(w101) -> ("Voltage (V)"=w100:dbl)
    n51 = Unbundle By Name(w104) -> ("Amp"=w109:dbl, "dt"=w108:dbl)
    n52 = local read "Output range"() -> (w106:cluster{"output high":dbl, "output low":dbl})
    n53 = call "Write To Measurement File2"("Signals"=w138, "Enable"=w153, "error in (no error)"=w154, "Filename"=w152) -> ("error out"=w151:errorcluster)  [unwired: 13 in, 2 out]
    n54 = call "PID.vi"("auto? (F)"="auto? (F)", "reinitialize? (F)"="reinitialize? (F)", "setpoint"="setpoint", "output range"=w106, "PID gains"="PID gains", "manual control"=w100, "dt (s)"=w108, "input"=w109) -> ("output"=w98:dbl)  [unwired: 3 in]
    "PID output" <- w98
    n55 = Merge Errors(w150, w151) -> (w149:errorcluster)
    n56 = local read "Waveform Config"() -> (w99:T8)
    n57 = local read "Sampling config"() -> (w96:cluster{"Fs":dbl, "#s":dbl})
    n58 = Bundle By Name(cluster=w99, "Voltage (V)"=w98) -> (w97:T8)
    n59 = call "Build Waveform.vi"("sampling config"=w96, "Config"=w97) -> ("Waveform"=w95:waveform(dbl))  [unwired: 8 in, 1 out]
    n60 = local write "Heater Modulation"(w95) -> ()
    n61 = Unbundle By Name(w149) -> ("status"=w145:bool)
  }
  n62 = while {
    tunnel: [w176] -> w76
    tunnel: [w172] -> w75
    tunnel: w71 -> [w175]
    tunnel: w72 -> [w174]
    tunnel: w25 -> [w171]
    tunnel: w24 -> [w170]
    tunnel: w2 -> [w169]
    tunnel: [w168] -> w22
    tunnel: [w166] -> w19
    tunnel: [w167] -> w18
    stop <- w177 stop-if-true
    n63 = call-poly <vilib>:"DAQmx Read.vi"("task/channels in"=w171, "error in"=w170) -> ("task out"=w168:refnum<k21>, "data"=w164:waveform(dbl)[], "error out"=w162:errorcluster)  [unwired: 11 in]
    n64 = local read "Heater Modulation"() -> (w163:waveform(dbl))
    n65 = call-poly <vilib>:"DAQmx Write.vi"("task/channels in"=w169, "auto start"=TRUE, "data"=w163, "error in"=w162) -> ("task out"=w167:refnum<k21>, "error out"=w166:errorcluster)  [unwired: 9 in, 1 out]
    n66 = Enqueue Element(queue=w175, element=w164, error in (no error)=w174) -> (queue out=w176:refnum<queue>, error out=w172:errorcluster)  [unwired: 1 in, 1 out]
    n67 = Compound Arithmetic op=OR(w166, w172, "Stop") -> (w177:bool)
  }
  n68 = call <vilib>:"DAQmx Stop Task.vi"("task/channels in"=w18, "error in"=w19) -> ("task out"=w20:refnum<k21>, "error out"=w21:errorcluster)  [unwired: 12 in]
  n69 = Flush Queue(queue=w76, error in (no error)=w75) -> (queue out=w77:refnum<queue>, error out=w78:errorcluster)  [unwired: 1 out]
  n70 = call <vilib>:"DAQmx Clear Task.vi"("task in"=w20, "error in"=w21) -> ("error out"=w10:errorcluster)  [unwired: 13 in]
  n71 = Release Queue(queue=w77, error in (no error)=w78) -> (error out=w74:errorcluster)  [unwired: 1 in, 2 out]
  n72 = call <vilib>:"DAQmx Stop Task.vi"("task/channels in"=w22, "error in"=w10) -> ("task out"=w82:refnum<k21>, "error out"=w83:errorcluster)  [unwired: 12 in]
  n73 = call <vilib>:"DAQmx Clear Task.vi"("task in"=w82, "error in"=w83) -> ("error out"=w23:errorcluster)  [unwired: 13 in]
  n74 = flat-sequence {
    tunnel: w23 -> [w182]
    tunnel: w74 -> [w181]
    tunnel: w70 -> [w178]
    frame #0 {
      w180 = T15 3 items=["no dialog", "OK message", "continue or stop message", "OK message + warnings", "continue/stop + warnings"] ("type of dialog (OK msg:1)")
      n75 = Merge Errors(w182, w181, w178) -> (w179:errorcluster)
      n76 = call <vilib>:"Simple Error Handler.vi"("type of dialog (OK msg:1)"=w180, "error in (no error)"=w179) -> ()  [unwired: 3 in, 5 out]
    }
  }
